vi "SMain.vi"() -> ()   [LabVIEW 2011] (continued)
                              i -> [w942]
                              n598 = Index Array(array=w945, index=w942) -> (element=w944:string)
                              n599 = Less?(x=w942, y=w943) -> (x < y?=w948:bool)
                              n600 = case shown="假" w948 {
                                tunnel: w947 -> [w950 w954]
                                tunnel: w946 -> [w949 w953]
                                tunnel: w944 -> [_ w952]
                                frame False {
                                n601 = property class="XYGraph (严格)"(reference=w950, "Value"=w949, "Caption.Visible"=FALSE ("标题.可见")) -> ()  [unwired: 1 in, 2 out]
                                }
                                frame True {
                                n602 = property class="XYGraph (严格)"(reference=w954, "Value"=w953, "Caption.Visible"=TRUE ("标题.可见"), "Caption.Text"=w952) -> ()  [unwired: 1 in, 2 out]
                                }
                              }
                            }
                            n603 = property on="Result" class="Str"("Visible"=TRUE ("可见"), "Text.Text"="Testing..." ("文本.文本"), "Text.TextColor"=u32 16860, "Text.FontSize"=u32 40 ("文本.字体:字号"), "Blinking"=FALSE ("闪烁")) -> ()  [unwired: 2 in, 2 out]
                          }
                          frame #3 {
                            n604 = local read "T Item Size"() -> (w980:i32)
                            n605 = local read "S Item Size"() -> (w981:i32)
                            n606 = local read "ILD Spec No"() -> (w973:i32)
                            n607 = local read "Urgent Stop"() -> (w969:bool)
                            n608 = Greater Than 0?(x=w980) -> (x > 0?=w979:bool)
                            n609 = Greater Than 0?(x=w981) -> (x > 0?=w978:bool)
                            n610 = Bundle("Demo"=w966, "Manual"=w965, "Urgent Stop"="Urgent Stop") -> (w968:T21)  [unwired: 1 in]
                            n611 = Or(x=w979, y=w978) -> (x .or. y?=w977:bool)
                            "Thru?" <- w977
                            n612 = case shown="真" w977 {
                              tunnel: w987 -> [_ w1009]
                              tunnel: w986 -> [_ w1008]
                              tunnel: w985 -> [_ w1007]
                              tunnel: w984 -> [_ w1006]
                              tunnel: w983 -> [_ w1005]
                              tunnel: w966 -> [_ w1004]
                              tunnel: w982 -> [_ w1003]
                              tunnel: w976 -> [_ w1002]
                              tunnel: w975 -> [_ w1001]
                              tunnel: [TRUE ("Total Reult") w1000] -> w974
                              tunnel: w973 -> [_ w999]
                              tunnel: ["" ("String data") w998] -> w972
                              tunnel: w971 -> [_ w997]
                              tunnel: w970 -> [_ w996]
                              tunnel: w969 -> [_ w995]
                              tunnel: w968 -> [_ w994]
                              tunnel: [bool[] [TRUE] ("Testing Results") w993] -> w964
                              tunnel: [string[] [] ("S-Para Item List") w992] -> w963
                              frame False {
                              }
                              frame True {
                                n613 = stacked-sequence {
                                seq-local: [_ _ _ w1069 _] -> [_ _ _ _ w1095]
                                tunnel: w1009 -> [w1021 _ _ _ _]
                                tunnel: w1008 -> [_ _ _ w1084 _]
                                tunnel: w1007 -> [_ _ _ w1074 _]
                                tunnel: w1006 -> [_ _ _ w1058 _]
                                tunnel: w1005 -> [w1031 _ _ _ _]
                                tunnel: w1004 -> [_ _ _ _ _]
                                tunnel: w1003 -> [_ _ _ w1057 _]
                                tunnel: w1002 -> [_ _ _ w1077 _]
                                tunnel: w1001 -> [_ _ _ _ _]
                                tunnel: [_ _ _ w1069 _] -> w1000
                                tunnel: w999 -> [_ _ _ w1076 _]
                                tunnel: [_ _ _ w1073 _] -> w998
                                tunnel: w997 -> [_ _ _ w1072 _]
                                tunnel: w996 -> [_ _ _ w1049 _]
                                tunnel: w995 -> [_ _ _ _ _]
                                tunnel: w994 -> [_ _ _ w1066 _]
                                tunnel: [_ _ _ w1061 _] -> w993
                                tunnel: [_ _ _ w1056 _] -> w992
                                frame #0 {
                                w1030 = u16 0 items=["Normal Input", "Start", "Product Inf", "End"] ("Summary Method")
                                # "一定要选第6项，StepImpedance\n20160926"
                                n614 = local read "Switch array"() -> (w1020:bool[][])
                                n615 = local read "Skew Spec(ps)"() -> (w1016:i32)
                                n616 = Bundle("DAQ Device"=w1021, "Switch array"=w1020, 0) -> (→"Matrix In":T22)  [unwired: 1 in]
                                n617 = local read "CMP setting"() -> (w1011:string)
                                n618 = Bundle("Start TimeNs"="Start TimeNs", "StopTimeNs"="StopTimeNs", "Data Points"="Data Points", "Compensation(ohm)"="Compensation(ohm)", "DataFormat"="DataFormat", "Impedance Filter"="Impedance Filter", "Filter Risetime(ps)"="Filter Risetime(ps)", "Impedance Spec String"="Impedance Spec String", "Skew Spec(ps)"=w1016, "CMP setting"=w1011) -> (→"TDR Setting":T12)  [unwired: 1 in]
                                n619 = call "Summary Generating.vi"("Summary Method"=w1030, "Status String"=w1031, "String 2"="S-parameter Testing....." ("Test Status:")) -> ()  [unwired: 25 in]
                                n620 = Format Date/Time String(time format string (%c)="%Y/%m/%d %H:%M:%S" ("时间格式字符串(%c)")) -> (date/time string=w1015:string)  [unwired: 2 in]
                                n621 = call <vilib>:"Trim Whitespace.vi"("string"=w1015) -> ("trimmed string"=w1013:string)  [unwired: 1 in]
                                n622 = Build Array(w1013) -> (w1012:string[])
                                n623 = local write "test time"(w1012) -> ()
                                }
                                frame #1 {
                                n624 = case shown="真" "Impedance Filter 2" {
                                selector: "Impedance Filter 2" -> [_ w1039]
                                frame False {
                                n625 = local read "TDR Setting"() -> (→"TDR Setting 2":T12)
                                }
                                frame True {
                                n626 = local read "DataFormat"() -> (w1040:i16)
                                n627 = local read "Skew Spec(ps) 2"() -> (w1036:i32)
                                n628 = Bundle("Start TimeNs 2"="Start TimeNs 2", "StopTimeNs 2"="StopTimeNs 2", "Data Points 2"="Data Points 2", "Compensation(ohm) 2"="Compensation(ohm) 2", "DataFormat"=w1040, w1039, "Filter Risetime(ps) 2"="Filter Risetime(ps) 2", "Impedance Spec String 2"="Impedance Spec String 2", "Skew Spec(ps) 2"=w1036, "") -> (w1035:T23)  [unwired: 1 in]
                                n629 = local write "TDR Setting 2"(w1035) -> ()
                                }
                                }
                                }
                                frame #2 {
                                n630 = local read "TDR Setting 2"() -> (w1046:T10)
                                n631 = local read "TDR Setting"() -> (w1047:T12)
                                n632 = Build Array(w1047, w1046) -> (→"TDR setting array":T6)
                                }
                                frame #3 {
                                n633 = local read "S-Para Item List"() -> (w1071:string[])
                                n634 = local read "TDR Test Item Name"() -> (w1070:string[])
                                n635 = local read "S-para Pair Name"() -> (w1055:string[])
                                n636 = local read "Length"() -> (w1054:string)
                                n637 = local read "Diff Test Item Name"() -> (w1053:string[])
                                n638 = local read "Diff Test Item smooth"() -> (w1052:string[])
                                n639 = local read "smooth point"() -> (w1051:i32)
                                n640 = local read "limitSpec"() -> (w1048:string[][])
                                n641 = Insert Into Array(array=w1071, new element=w1070) -> (w1056:string[])  [unwired: 1 in]
                                "itemList" <- w1056
                                n642 = Bundle By Name(cluster="Information In", "Sample PN:"=w1058, "SampleSN:"=w1057, "Sparam Test Item"=w1056, "S-para Pair Name"=w1055, "Length"=w1054, "Diff Test Item Name"=w1053, "Diff Test Item Name smooth"=w1052, "smooth point"=w1051, "limitSpec"=w1048) -> (w1050:T4)
                                n643 = local read "Reference"() -> (w1065:T5)
                                n644 = local read "proBar_ref"() -> (w1062:refnum<vi>)
                                n645 = local read "TDR setting array"() -> (w1060:T6)
                                n646 = local read "Option"() -> (w1067:T11)
                                n647 = local read "Matrix In"() -> (w1079:T13)
                                n648 = local read "2X IL"() -> (w1068:dbl[])
                                n649 = call "Sparameter Testing.vi"("VNA Model:"=w1074, "VNA VISA"=w1084, "Port Type"=w1077, "Reference"=w1065, "VISA COM"=w1072, "Information In"=w1050, "TDR setting array"=w1060, "Mode(Demo,Manual)"=w1066, "DAQ  Model:"=w1049, "S4P Data Type"=enum16{"THRU", "NEXT", "FEXT"}."THRU", "Matrix  In"=w1079, "ILDSpec"=w1076, "Option"=w1067, "MulChannel?"="By Channel?", "2X Thru"=w1068, "proBar_ref"=w1062) -> ("String data"=w1073:string, "Basic Path"=→"original Path":path, "Frequency(Hz)"=→"Frequency(Hz)":dbl[], "Data Out"=→"Data Out":dbl[][][], "Testing Results"=w1061:bool[], "Total Reult"=w1069:bool, "TXT Data Path"=→"TXT Data Path":path, "Items Result"=→"Items Result":string[], "S4P Data Path"=→"S4P Data Path":path)  [unwired: 2 in, 1 out]
                                }
                                frame #4 {
                                n650 = local read "S-Para Item List"() -> (w1100:string[])
                                n651 = local read "TDR Test Item Name"() -> (w1085:string[])
                                n652 = local read "Items Result"() -> (w1101:string[])
                                n653 = Array Size(array=w1100) -> (size(s)=w1099:i32)
                                n654 = Split 1D Array(array=w1101, index=w1099) -> (first subarray=w1098:string[], second subarray=w1088:string[])
                                n655 = Search 1D Array(1D array=w1085, element="Pskew" ("元素")) -> (index of element=w1087:i32)  [unwired: 1 in]
                                n656 = Not Equal?(x=w1087, y=-1) -> (x != y?=w1089:bool)
                                n657 = case shown="真" w1089 {
                                tunnel: w1088 -> [w1102 w1106]
                                tunnel: w1087 -> [_ w1105]
                                tunnel: [w1102 w1103] -> w1086
                                frame False {
                                }
                                frame True {
                                n658 = Delete From Array(array=w1106, length=1 ("长度"), index=w1105) -> (array with subset deleted=w1103:string[])  [unwired: 1 out]
                                }
                                }
                                n659 = Select(t="PASS" ("字符串"), s=w1095, f="FAIL" ("字符串")) -> (s? t:f=w1093:string)
                                n660 = Insert Into Array(array=w1086, new element=w1098) -> (w1094:string[])  [unwired: 1 in]
                                n661 = Insert Into Array(array=w1094, new element=w1093) -> (w1092:string[])  [unwired: 1 in]
                                n662 = local write "Items Result"(w1092) -> ()
                                }
                                }
                              }
                            }
                            "SparaReult" <- w974
                            "Thru String data" <- w972
                            "SparaReults" <- w964
                            "SparaLists" <- w963
                          }
                          frame #4 {
                            n663 = local read "Diff Test Item Name"() -> (w1120:string[])
                            n664 = local read "Urgent Stop"() -> (w1113:bool)
                            n665 = local read "limitSpec"() -> (w1107:string[][])
                            n666 = local read "NEXT Pair Name"() -> (w1130:string[])
                            n667 = Bundle("Demo"=w1111, "Manual"=w1110, "Urgent Stop"=w1113) -> (w1112:T21)  [unwired: 1 in]
                            n668 = Search 1D Array(1D array=w1120, element="NEXT" ("元素")) -> (index of element=w1129:i32)  [unwired: 1 in]
                            n669 = local read "Urgent Stop"() -> (w1115:bool)
                            n670 = Not Equal?(x=w1129, y=-1) -> (x != y?=w1131:bool)
                            "NEXT?" <- w1131
                            n671 = case shown="真" w1131 {
                              tunnel: w1130 -> [_ w1157]
                              tunnel: w1107 -> [_ w1156]
                              tunnel: w1122 -> [_ w1155]
                              tunnel: w1129 -> [_ w1154]
                              tunnel: w1128 -> [_ w1153]
                              tunnel: w1127 -> [_ w1152]
                              tunnel: w1126 -> [_ w1151]
                              tunnel: w1125 -> [_ w1150]
                              tunnel: w1124 -> [_ w1149]
                              tunnel: w1123 -> [_ w1148]
                              tunnel: w1121 -> [_ w1147]
                              tunnel: w1120 -> [_ w1146]
                              tunnel: [TRUE ("Total Reult") w1145] -> w1119
                              tunnel: [_ w1144] -> w1118
                              tunnel: w1117 -> [_ w1143]
                              tunnel: w1116 -> [_ w1142]
                              tunnel: w1115 -> [_ w1141]
                              tunnel: w1114 -> [_ w1140]
                              tunnel: w1112 -> [_ w1139]
                              tunnel: [string[] [] ("NEXT Pair Name") w1138] -> w1109
                              tunnel: [bool[] [TRUE] ("Testing Results") w1137] -> w1108
                              frame False {
                              }
                              frame True {
                                n672 = stacked-sequence {
                                seq-local: [_ w1193] -> [_ _]
                                tunnel: w1157 -> [w1159 _]
                                tunnel: w1156 -> [w1160 _]
                                tunnel: w1155 -> [_ _]
                                tunnel: w1154 -> [_ _]
                                tunnel: w1153 -> [w1175 _]
                                tunnel: w1152 -> [_ w1199]
                                tunnel: w1151 -> [_ w1200]
                                tunnel: w1150 -> [w1167 _]
                                tunnel: w1149 -> [w1179 _]
                                tunnel: w1148 -> [w1166 _]
                                tunnel: w1147 -> [_ w1198]
                                tunnel: w1146 -> [w1163 _]
                                tunnel: [_ w1193] -> w1145
                                tunnel: [_ w1197] -> w1144
                                tunnel: w1143 -> [_ w1196]
                                tunnel: w1142 -> [_ w1195]
                                tunnel: w1141 -> [_ _]
                                tunnel: w1140 -> [_ _]
                                tunnel: w1139 -> [_ w1191]
                                tunnel: [_ w1189] -> w1138
                                tunnel: [_ w1188] -> w1137
                                frame #0 {
                                w1169 = "MDNEXT" ("元素")
                                w1181 = u16 0 items=["Normal Input", "Start", "Product Inf", "End"] ("Summary Method")
                                n673 = local read "Diff Test Item smooth"() -> (w1162:string[])
                                n674 = Build Array("NEXT" ("元素")) -> (w1170:string[])
                                n675 = local read "Length"() -> (w1164:string)
                                n676 = Search 1D Array(1D array=w1163, element=w1169) -> (index of element=w1173:i32)  [unwired: 1 in]
                                n677 = Not Equal?(x=w1173, y=-1) -> (x != y?=w1171:bool)
                                n678 = case shown="真" w1171 {
                                tunnel: w1170 -> [w1182 w1185]
                                tunnel: w1169 -> [_ w1184]
                                tunnel: [w1182 w1183] -> w1165
                                frame False {
                                }
                                frame True {
                                n679 = Build Array (concatenate)(w1185, w1184) -> (w1183:string[])
                                }
                                }
                                "NEXTList" <- w1165
                                n680 = local read "smooth point"() -> (w1161:i32)
                                n681 = call "Summary Generating.vi"("Summary Method"=w1181, "Status String"=w1179, "String 2"="NEXT Testing....." ("Test Status:")) -> ()  [unwired: 25 in]
                                n682 = local read "Switch array"() -> (w1176:bool[][])
                                n683 = local read "S-Pair Loop"() -> (w1177:i32)
                                n684 = Bundle("DAQ Device"=w1175, "Switch array"=w1176, "S-Pair Loop"=w1177) -> (w1174:T24)  [unwired: 1 in]
                                n685 = local write "Matrix In"(w1174) -> ()
                                n686 = Bundle By Name(cluster="Information In 2", "Sample PN:"=w1167, "SampleSN:"=w1166, "Sparam Test Item"=w1165, "S-para Pair Name"=w1159, "Length"=w1164, "Diff Test Item Name"=w1163, "Diff Test Item Name smooth"=w1162, "smooth point"=w1161, "limitSpec"=w1160) -> (→"NEXT INF":T4)
                                }
                                frame #1 {
                                n687 = local read "NEXT INF"() -> (w1186:T4)
                                n688 = local read "proBar_ref"() -> (w1190:refnum<vi>)
                                n689 = local read "Reference"() -> (w1187:T5)
                                n690 = local read "Matrix In"() -> (w1202:T13)
                                n691 = local read "Option"() -> (w1192:T11)
                                n692 = call "Sparameter Testing.vi"("VNA Model:"=w1200, "VNA VISA"=w1199, "Port Type"=w1198, "Reference"=w1187, "VISA COM"=w1196, "Information In"=w1186, "Mode(Demo,Manual)"=w1191, "DAQ  Model:"=w1195, "S4P Data Type"=enum16{"THRU", "NEXT", "FEXT"}."NEXT", "Matrix  In"=w1202, "Option"=w1192, "proBar_ref"=w1190) -> ("String data"=w1197:string, "Testing Results"=w1188:bool[], "Total Reult"=w1193:bool, "Items Result"=→"NEXT Result":string[])  [unwired: 6 in, 6 out]
                                n693 = Unbundle By Name(w1186) -> ("S-para Pair Name"=w1189:string[])
                                }
                                }
                              }
                            }
                            "NEXTReult" <- w1119
                            "NEXT String data" <- w1118
                            "NEXTList" <- w1109
                            "NEXTReults" <- w1108
                          }
                          frame #5 {
                            n694 = local read "Diff Test Item Name"() -> (w1214:string[])
                            n695 = local read "limitSpec"() -> (w1204:string[][])
                            n696 = local read "Urgent Stop"() -> (w1208:bool)
                            n697 = local read "FEXT Pair Name"() -> (w1215:string[])
                            n698 = Search 1D Array(1D array=w1214, element="FEXT" ("元素")) -> (index of element=w1224:i32)  [unwired: 1 in]
                            n699 = Bundle("Demo"=w1206, "Manual"=w1205, "Urgent Stop"=w1208) -> (w1207:T21)  [unwired: 1 in]
                            n700 = Not Equal?(x=w1224, y=-1) -> (x != y?=w1225:bool)
                            "FEXT?" <- w1225
                            n701 = case shown="真" w1225 {
                              tunnel: w1215 -> [_ w1248]
                              tunnel: w1204 -> [_ w1247]
                              tunnel: w1217 -> [_ w1246]
                              tunnel: w1224 -> [_ w1245]
                              tunnel: w1223 -> [_ w1244]
                              tunnel: w1222 -> [_ w1243]
                              tunnel: w1221 -> [_ w1242]
                              tunnel: w1220 -> [_ w1241]
                              tunnel: w1219 -> [_ w1240]
                              tunnel: w1206 -> [_ w1239]
                              tunnel: w1218 -> [_ w1238]
                              tunnel: w1216 -> [_ w1237]
                              tunnel: w1214 -> [_ w1236]
                              tunnel: [TRUE ("Total Reult") w1235] -> w1213
                              tunnel: [_ w1234] -> w1212
                              tunnel: w1211 -> [_ w1233]
                              tunnel: w1210 -> [_ w1232]
                              tunnel: w1209 -> [_ w1231]
                              tunnel: w1207 -> [_ w1230]
                              tunnel: [_ w1229] -> w1203
                              frame False {
                              }
                              frame True {
                                n702 = stacked-sequence {
                                seq-local: [_ w1284 _] -> [_ _ _]
                                tunnel: w1248 -> [w1255 _ _]
                                tunnel: w1247 -> [w1250 _ _]
                                tunnel: w1246 -> [_ _ _]
                                tunnel: w1245 -> [_ _ _]
                                tunnel: w1244 -> [w1269 _ _]
                                tunnel: w1243 -> [_ w1291 _]
                                tunnel: w1242 -> [_ w1292 _]
                                tunnel: w1241 -> [w1258 _ _]
                                tunnel: w1240 -> [w1272 _ _]
                                tunnel: w1239 -> [_ _ _]
                                tunnel: w1238 -> [w1257 _ _]
                                tunnel: w1237 -> [_ w1290 _]
                                tunnel: w1236 -> [w1253 _ _]
                                tunnel: [_ w1284 _] -> w1235
                                tunnel: [_ w1288 _] -> w1234
                                tunnel: w1233 -> [_ w1287 _]
                                tunnel: w1232 -> [_ w1286 _]
                                tunnel: w1231 -> [_ _ _]
                                tunnel: w1230 -> [_ w1282 _]
                                tunnel: [_ w1279 _] -> w1229
                                frame #0 {
                                w1260 = "MDFEXT" ("元素")
                                w1274 = u16 0 items=["Normal Input", "Start", "Product Inf", "End"] ("Summary Method")
                                n703 = local read "Diff Test Item smooth"() -> (w1252:string[])
                                n704 = local read "smooth point"() -> (w1251:i32)
                                n705 = Search 1D Array(1D array=w1253, element=w1260) -> (index of element=w1264:i32)  [unwired: 1 in]
                                n706 = Not Equal?(x=w1264, y=-1) -> (x != y?=w1262:bool)
                                n707 = Build Array("FEXT" ("元素")) -> (w1261:string[])
                                n708 = case shown="假" w1262 {
                                tunnel: w1261 -> [w1275 w1278]
                                tunnel: w1260 -> [_ w1277]
                                tunnel: [w1275 w1276] -> w1256
                                frame False {
                                }
                                frame True {
                                n709 = Build Array (concatenate)(w1278, w1277) -> (w1276:string[])
                                }
                                }
                                "FEXTLIst" <- w1256
                                n710 = call "Summary Generating.vi"("Summary Method"=w1274, "Status String"=w1272, "String 2"="FEXT Testing....." ("Test Status:")) -> ()  [unwired: 25 in]
                                n711 = local read "S-Pair Loop"() -> (w1266:i32)
                                n712 = local read "N-Pair Loop"() -> (w1267:i32)
                                n713 = local read "Switch array"() -> (w1270:bool[][])
                                n714 = local read "Length"() -> (w1254:string)
                                n715 = Add(x=w1266, y=w1267) -> (x+y=w1265:i32)
                                n716 = Bundle("DAQ Device"=w1269, "Switch array"=w1270, w1265) -> (w1268:T22)  [unwired: 1 in]
                                n717 = Bundle By Name(cluster=T4 {"Sample PN: "="", "SampleSN:"="", "Sparam Test Item"=[], "S-para Pair Name"=[], "Length"="", "Diff Test Item Name"=["SDD21", "SDD22", "SCD21", "SCD22", "SCC11", "NEXT", "FEXT"], "Diff Test Item Name smooth"=[], "smooth point"=0.0, "limitSpec"=[], "switchIndexOffset"=0.0, "testType"=enum."Loss"} ("Information In 3"), "Sample PN:"=w1258, "SampleSN:"=w1257, "Sparam Test Item"=w1256, "S-para Pair Name"=w1255, "Length"=w1254, "Diff Test Item Name"=w1253, "Diff Test Item Name smooth"=w1252, "smooth point"=w1251, "limitSpec"=w1250) -> (→"FEXT INF":T4)
                                n718 = local write "Matrix In"(w1268) -> ()
                                }
                                frame #1 {
                                n719 = local read "FEXT INF"() -> (w1280:T4)
                                n720 = local read "Reference"() -> (w1289:T5)
                                n721 = local read "proBar_ref"() -> (w1281:refnum<vi>)
                                n722 = local read "Matrix In"() -> (w1294:T13)
                                n723 = local read "Option"() -> (w1283:T11)
                                n724 = call "Sparameter Testing.vi"("VNA Model:"=w1292, "VNA VISA"=w1291, "Port Type"=w1290, "Reference"=w1289, "VISA COM"=w1287, "Information In"=w1280, "Mode(Demo,Manual)"=w1282, "DAQ  Model:"=w1286, "S4P Data Type"=enum16{"THRU", "NEXT", "FEXT"}."FEXT", "Matrix  In"=w1294, "Option"=w1283, "proBar_ref"=w1281) -> ("String data"=w1288:string, "Testing Results"=w1279:bool[], "Total Reult"=w1284:bool, "Items Result"=→"FEXT Result":string[])  [unwired: 6 in, 6 out]
                                }
                                frame #2 {
                                }
                                }
                              }
                            }
                            "FEXTReult" <- w1213
                            "FEXT String data" <- w1212
                            "FEXT Results" <- w1203
                          }
                          frame #6 {
                            # "save general"
                            n725 = local read "VNA Model:"() -> (w1302:enum16{"E5071C", "N5230A(C)", "N5224A"})
                            n726 = property on="Approval:" class="Ring (严格)"() -> ("RingText.Text"=w1305:string)  [unwired: 2 in, 2 out]
                            n727 = property on="Tester:" class="Ring (严格)"() -> ("RingText.Text"=w1306:string)  [unwired: 2 in, 2 out]
                            n728 = local read "NEXTList"() -> (w1317:string[])
                            n729 = local read "SparaReults"() -> (w1314:bool[])
                            n730 = local read "itemList"() -> (w1318:string[])
                            n731 = local read "NEXTReults"() -> (w1313:bool[])
                            n732 = local read "FEXT Results"() -> (w1312:bool[])
                            n733 = local read "FEXTLIst"() -> (w1316:string[])
                            n734 = local read "Applicant:"() -> (w1309:string)
                            n735 = local read "PN Des"() -> (w1308:string)
                            n736 = local read "Report No."() -> (w1304:string)
                            n737 = local read "P/N:"() -> (w1307:string)
                            n738 = local read "Sample #"() -> (w1303:string)
                            n739 = Insert Into Array(array=w1314, new element #1=w1313, new element #2=w1312) -> (w1311:bool[])  [unwired: 1 in]
                            n740 = Insert Into Array(array=w1318, new element #1=w1317, new element #2=w1316) -> (w1315:string[])  [unwired: 1 in]
                            n741 = call "getReportMsg.vi"("partDescription"=w1308, "partNo"=w1307, "fixtureSerialNo"="Fixture No", "preparedBy"=w1306, "approvedBy"=w1305, "temprature"="Temperature(℃)", "VNA Model:"=w1302, "reportNo"=w1304, "application"=w1309, "sampleNo"=w1303, "rHumidity"="Relative Humidity(%)") -> ("value"=w1300:string[], "item"=w1301:string[])  [unwired: 7 in]
                            n742 = for {
                              tunnel: w1311 -> [w1322] mode=indexing
                              tunnel: [w1319] -> w1310 mode=indexing
                              n743 = Select(t="Pass", s=w1322, f="Fail") -> (s? t:f=w1319:string)
                            }
                            n744 = local read "TXT Data Path"() -> (w1296:path)
                            n745 = call "saveGeneral.vi"("itemList"=w1315, "resultsStr"=w1310, "item"=w1301, "文件（使用对话框）"=w1296, "value"=w1300) -> ("cluResult"=→"cluResult":T2)  [unwired: 6 in, 4 out]
                          }
                          frame #7 {
                            n746 = case shown="假" w1323 {
                              tunnel: [w1334 w1337] -> w1328
                              frame False {
                                n747 = local read "original Path"() -> (w1336:path)
                                n748 = Build Path(base path=w1336, name or relative path="TXT" ("名称或相对路径")) -> (appended path=w1334:path)
                              }
                              frame True {
                                n749 = call <vilib>:"Application Directory.vi"() -> ("Application Directory"=w1339:path)
                                n750 = Build Path(base path=w1339, name or relative path="Demo_data") -> (appended path=w1337:path)
                              }
                            }
                            n751 = local read "S-para Pair Name"() -> (w1329:string[])
                            n752 = local read "S-Para Item List"() -> (w1330:string[])
                            n753 = local read "frePoints"() -> (w1327:string[])
                            n754 = call "采集频点值.vi"("频率点（MHZ）"=w1327, "测试对名称"=w1329, "S参数测试项目"=w1330, "TXT文件所处路径"=w1328) -> ("测试项目及频点在DB输出"=w1325:string, "测试项目及频点在txt输出"=→"测试项目及频点在txt输出":string)
                            n755 = control-ref of="db_ResultString"() -> (w1333:refnum<vi>)
                            n756 = property class="Str"(reference=w1333) -> (reference out=w1324:refnum<vi>, "Value"=w1332:string)  [unwired: 1 in, 1 out]
                            n757 = Concatenate Strings(w1332, w1325) -> (w1331:string)
                            n758 = property class="Str"(reference=w1324, "Value"=w1331) -> ()  [unwired: 1 in, 2 out]
                          }
                          frame #8 {
                            # "烧录、检验EEPROM"
                            n759 = local read "EEPROMTF"() -> (w1342:bool)
                            n760 = local read "EE Write"() -> (w1341:bool)
                            n761 = And(x=w1342, y=w1341) -> (x .and. y?=w1340:bool)
                            n762 = case shown="真" w1340 {
                              tunnel: w1343 -> [w1348 w1374]
                              frame False {
                                n763 = property class="Str"(reference=w1348) -> (reference out=w1344:refnum<vi>, "Value"=w1347:string)  [unwired: 1 in, 1 out]
                                n764 = local write "EEResult"(TRUE ("EEResult")) -> ()
                                n765 = Concatenate Strings(w1347, "\nEEPROM write option not selected：EEPROM need not burn\n" ("字符串")) -> (w1346:string)
                                n766 = property class="Str"(reference=w1344, "Value"=w1346) -> ()  [unwired: 1 in, 2 out]
                              }
                              frame True {
                                w1353 = "\n"
                                n767 = local read "mid_str_labelType"() -> (w1371:string)
                                n768 = local read "PN description"() -> (w1351:string)
                                n769 = local read "RS232 I2C VISA"() -> (w1373:refnum<visa-resource-name>)
                                n770 = local read "mid_array_temp_int"() -> (w1366:u8[][])
                                n771 = local read "Adaptor:"() -> (w1372:enum16{"RS232 - IIC", "LUXSHARE - IIC"})
                                n772 = Concatenate Strings(w1371, w1351) -> (w1368:string)
                                n773 = property class="Str"(reference=w1374) -> (reference out=w1355:refnum<vi>, "Value"=w1362:string)  [unwired: 1 in, 1 out]
                                n774 = call "readLabelTypeForH3C.vi"("input_str_labelType"=w1368) -> ("show_str_011string"=w1350:string)  [unwired: 1 out]
                                n775 = flat-sequence {
                                tunnel: w1373 -> [w1378]
                                tunnel: w1372 -> [w1379]
                                tunnel: w1366 -> [w1381]
                                tunnel: w1350 -> [w1380]
                                tunnel: [w1379] -> w1370
                                tunnel: [w1378] -> w1369
                                tunnel: w1368 -> [w1377]
                                tunnel: [w1377] -> w1367
                                tunnel: w1366 -> [w1376]
                                tunnel: [w1376] -> w1365
                                tunnel: ["Write EEprom"] -> w1354
                                tunnel: w1370 -> [w1388]
                                tunnel: w1369 -> [w1387]
                                tunnel: w1367 -> [w1386]
                                tunnel: w1365 -> [w1384]
                                tunnel: [w1385] -> w1364
                                tunnel: [w1384] -> w1363
                                tunnel: [w1383] -> w1358
                                tunnel: ["Read EEprom"] -> w1352
                                tunnel: w1364 -> [w1391]
                                tunnel: w1363 -> [w1393]
                                tunnel: [w1392] -> w1361
                                tunnel: [w1391] -> w1360
                                tunnel: [w1390] -> w1359
                                tunnel: w1358 -> [w1389]
                                tunnel: [w1389] -> w1357
                                tunnel: w1360 -> [w1402]
                                tunnel: w1359 -> [w1400]
                                tunnel: w1357 -> [w1401]
                                tunnel: w1356 -> [w1403]
                                tunnel: w1355 -> [w1404]
                                frame #0 {
                                n776 = call "EEPROM烧录模块.vi"("input_array_temp_int"=w1381, "input_str_011string"=w1380, "Visa Port :"=w1378, "Adaptor:"=w1379) -> ()  [unwired: 6 in, 2 out]
                                }
                                frame #1 {
                                n777 = call "EEPROM读取模块.vi"("input_array_temp_int"=w1384, "input_str_labelType"=w1386, "VISA :"=w1387, "Adaptor"=w1388) -> ("pagesEqual00?"=w1383:bool, "show_array_read_int"=w1385:u8[][])  [unwired: 6 in]
                                }
                                frame #2 {
                                n778 = call "compareTempAndRead.vi"("input_array_temp"=w1393, "input_array_read"=w1391) -> ("show_str_message"=w1392:string, "show_testResult"=w1390:bool)  [unwired: 8 in]
                                }
                                frame #3 {
                                n779 = local read "original Path"() -> (w1397:path)
                                n780 = local read "Demo"() -> (w1398:bool)
                                n781 = And(x=w1401, y=w1400) -> (x .and. y?=→"EEResult":bool)
                                n782 = Build Path(base path=w1397, name or relative path="TXT" ("名称或相对路径")) -> (appended path=w1396:path)
                                n783 = Select(t=w1397, s=w1398, f=w1396) -> (s? t:f=w1395:path)
                                n784 = call "saveEEPFiles2.vi"("input_path"=w1395, "input_array_read_int"=w1402) -> ()  [unwired: 10 in]
                                }
                                frame #4 {
                                n785 = property class="Str"(reference=w1404, "Value"=w1403) -> ()  [unwired: 1 in, 2 out]
                                }
                                }
                                n786 = Concatenate Strings(w1362, w1353, w1354, w1353, w1352, w1353, w1361) -> (w1356:string)
                              }
                            }
                          }
                          frame #9 {
                            # "打印标签"
                            n787 = Not(x=w1405) -> (.not. x?=w1406:bool)
                            n788 = case shown="假" w1406 {
                              tunnel: w1407 -> [w1419 w1487]
                              frame True {
                                (unwired) "0. P/N  luxshare\n1. AWG\n2. Length（不可用）\n3. SN\n4. Custmer PN "  # Data In Format
                                n789 = local read "SparaReult"() -> (w1416:bool)
                                n790 = local read "NEXTReult"() -> (w1415:bool)
                                n791 = local read "FEXTReult"() -> (w1414:bool)
                                n792 = local read "EEResult"() -> (w1412:bool)
                                n793 = local read "LabelTF"() -> (w1413:bool)
                                n794 = local write "proBar"(u8 96 ("proBar")) -> ()
                                n795 = Compound Arithmetic op=AND(w1412, w1416, w1415, w1414, w1413) -> (w1410:bool)
                                n796 = property class="Str"(reference=w1419) -> (reference out=w1418:refnum<vi>, "Value"=w1417:string)  [unwired: 1 in, 1 out]
                                n797 = Or(x=w1410, y=FALSE) -> (x .or. y?=w1408:bool)
                                n798 = case shown="真" w1408 {
                                tunnel: w1418 -> [w1421 w1425]
                                tunnel: w1417 -> [w1423 w1426]
                                frame False {
                                n799 = Concatenate Strings(w1423, "\nNo Label has been printed!\n") -> (w1420:string)
                                n800 = property class="Str"(reference=w1421, "Value"=w1420) -> ()  [unwired: 1 in, 2 out]
                                n801 = local write "条码输出"("nolabel" ("条码输出")) -> ()
                                }
                                frame True {
                                n802 = stacked-sequence {
                                seq-local: [w1428 _ _ _] -> [_ w1439 _ _]
                                seq-local: [_ w1438 _ _] -> [_ _ w1463 _]
                                tunnel: w1426 -> [w1430 _ _ _]
                                tunnel: w1425 -> [w1427 w1436 w1464 _]
                                frame #0 {
                                n803 = Concatenate Strings(w1430, "\nLabel Printe Command Was Sent. \n") -> (w1428:string)
                                n804 = property class="Str"(reference=w1427, "Value"=w1428) -> ()  [unwired: 1 in, 2 out]
                                }
                                frame #1 {
                                n805 = vi-ref "打标签模式选择.vi"() -> (w1448:refnum<vi>)
                                n806 = property class="VI"(reference=w1448) -> ("Name"=w1447:string)  [unwired: 1 in, 2 out]
                                n807 = local read "midVar_time_date"() -> (w1456:timestamp)
                                n808 = local read "midVar_str_SN"() -> (w1457:string)
                                n809 = local read "Printer VISA"() -> (w1453:refnum<visa-resource-name>)
                                n810 = local read "Label Type"() -> (w1455:string[])
                                n811 = local read "LabelNum"() -> (w1452:i32)
                                n812 = local read "Data In"() -> (w1454:string[])
                                n813 = Open VI Reference(type specifier VI Refnum (for type only)=refnum<vi> refnum ("类型说明符VI引用句柄（仅用于类型）"), vi path=w1447, options=128 ("选项")) -> (vi reference=w1444:refnum<vi>, error out=w1440:errorcluster)  [unwired: 3 in]
                                n814 = local read "打印模式"() -> (w1451:enum16{"IT Print", "EE Print"})
                                n815 = local read "PRINT"() -> (w1449:refnum<k24>)
                                n816 = local read "SN"() -> (w1450:refnum<k24>)
                                n817 = call-by-ref "Start Asynchronous Call"(reference=w1444, error in=w1440, "LabelNum"=w1452, "Printer VISA"=w1453, "Data In"=w1454, "Label Type"=w1455, "midVar_time_date"=w1456, "打印模式"=w1451, "midVar_str_SN"=w1457, "引用"=w1450, "print path local"="Fast Print", "PRINT"=w1449, "错误输入（无错误）"="错误输入（无错误）", "条码类型"="制程条码") -> (reference out=w1442:refnum<vi>, error out=w1435:errorcluster)  [unwired: 4 in, 4 out]
                                n818 = flat-sequence {
                                tunnel: w1442 -> [w1458]
                                tunnel: [w1458] -> w1441
                                frame #0 {
                                n819 = Wait (ms)(milliseconds to wait=u32 1500 ("等待时间（毫秒）")) -> ()  [unwired: 1 out]
                                }
                                }
                                n820 = Unbundle(w1435) -> ("source"=w1434:string)  [unwired: 2 out]
                                n821 = local write "labelFlag"(TRUE ("labelFlag")) -> ()
                                n822 = Concatenate Strings(w1439, w1434, "\n") -> (w1438:string)
                                n823 = Close Reference(reference=w1441) -> ()  [unwired: 1 in, 1 out]
                                n824 = property class="Str"(reference=w1436, "Value"=w1438) -> ()  [unwired: 1 in, 2 out]
                                }
                                frame #2 {
                                n825 = local read "S/N:"() -> (w1462:string)
                                n826 = Concatenate Strings(w1462, " :Test Finished !" ("字符串")) -> (w1460:string)
                                n827 = Concatenate Strings(w1463, "\nLabel has been printed!\n", w1460) -> (w1465:string)
                                n828 = property class="Str"(reference=w1464, "Value"=w1465) -> ()  [unwired: 1 in, 2 out]
                                }
                                frame #3 {
                                n829 = local read "P/N:"() -> (w1474:string)
                                n830 = local read "Impedance Spec String"() -> (w1469:string)
                                n831 = local read "Current Testing Label/当前测试条码"() -> (w1473:string)
                                n832 = local read "original Path"() -> (w1472:path)
                                n833 = Build Path(base path=w1472, name or relative path="TXT" ("名称或相对路径")) -> (appended path=w1470:path)
                                n834 = call "TDD一致性检查.vi"("TDD filePath"=w1470, "Spec String"=w1469, "SN"=w1473, "PN"=w1474) -> ("报警颜色"=w1467:string, "判定"=w1468:bool)  [unwired: 6 in]
                                n835 = case shown="假" w1468 {
                                tunnel: w1467 -> [w1476 _]
                                frame False {
                                n836 = control-ref of="Test Status:"() -> (w1477:refnum<vi>)
                                n837 = call "颜色常量（汉字）.vi"("颜色"=w1476) -> ("颜色常量"=w1475:u32)  [unwired: 10 in]
                                n838 = property on="属性节点" class="Str"(reference=w1477, "Text.BGColor"=w1475, "Text.TextColor"=u32 0) -> ()  [unwired: 1 in, 2 out]
                                }
                                frame True {
                                }
                                }
                                }
                                }
                                }
                                }
                              }
                              frame False {
                                (unwired) "0. P/N  luxshare\n1. AWG\n2. Length（不可用）\n3. SN\n4. Custmer PN "  # Data In Format
                                n839 = local write "proBar"(u8 96 ("proBar")) -> ()
                                n840 = property class="Str"(reference=w1487) -> (reference out=w1483:refnum<vi>, "Value"=w1486:string)  [unwired: 1 in, 1 out]
                                n841 = local read "S/N:"() -> (w1481:string)
                                n842 = disable-structure shown="禁用" {
                                frame Disabled {
                                n843 = local read "midVar_time_date"() -> (w1496:timestamp)
                                n844 = local read "midVar_str_SN"() -> (w1495:string)
                                n845 = local read "Printer VISA"() -> (w1491:refnum<visa-resource-name>)
                                n846 = local read "Label Type"() -> (w1497:string[])
                                n847 = local read "LabelNum"() -> (w1499:i32)
                                n848 = local read "Data In"() -> (w1498:string[])
                                n849 = local read "PRINT"() -> (w1489:refnum<k24>)
                                n850 = local read "SN"() -> (w1488:refnum<k24>)
                                n851 = local read "打印模式"() -> (w1494:enum16{"IT Print", "EE Print"})
                                n852 = call "打标签模式选择.vi"("LabelNum"=w1499, "Printer VISA"=w1491, "Data In"=w1498, "Label Type"=w1497, "midVar_time_date"=w1496, "打印模式"=w1494, "midVar_str_SN"=w1495, "引用"=w1488, "print path local"=TRUE, "PRINT"=w1489) -> ("labelFlag"=w1493:bool, "条码输出"=w1492:string)  [unwired: 6 in, 2 out]
                                n853 = local write "labelFlag"(w1493) -> ()
                                n854 = local write "条码输出"(w1492) -> ()
                                }
                                frame Enabled {
                                }
                                }
                                n855 = Concatenate Strings(w1481, " :Test Finished !" ("字符串")) -> (w1479:string)
                                n856 = Concatenate Strings(w1486, "\nDemo mode Label has been printed!\n", w1479) -> (w1482:string)
                                n857 = property class="Str"(reference=w1483, "Value"=w1482) -> ()  [unwired: 1 in, 2 out]
                              }
                            }
                          }
                          frame #10 {
                            n858 = property class="Str"(reference=w1503) -> ("Value"=w1502:string)  [unwired: 1 in, 2 out]